vi "AeroQuadConfigurator.vi"() -> ()   [LabVIEW 2010] (continued)
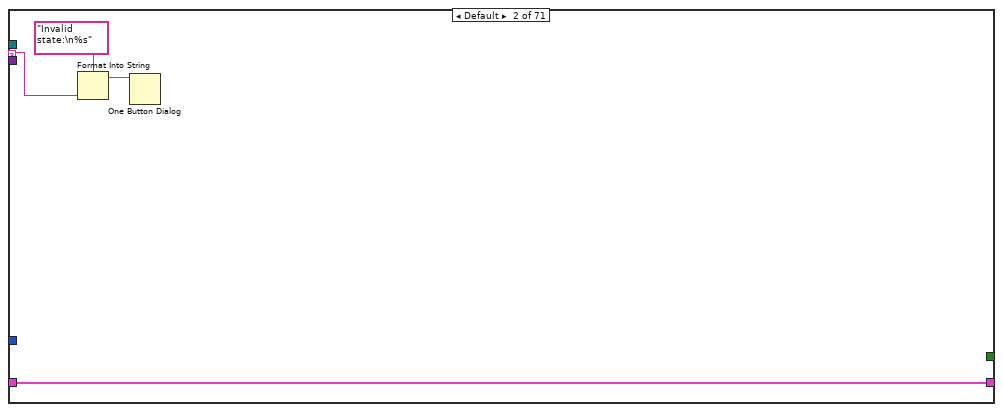
[diagram p3: hidden frame]
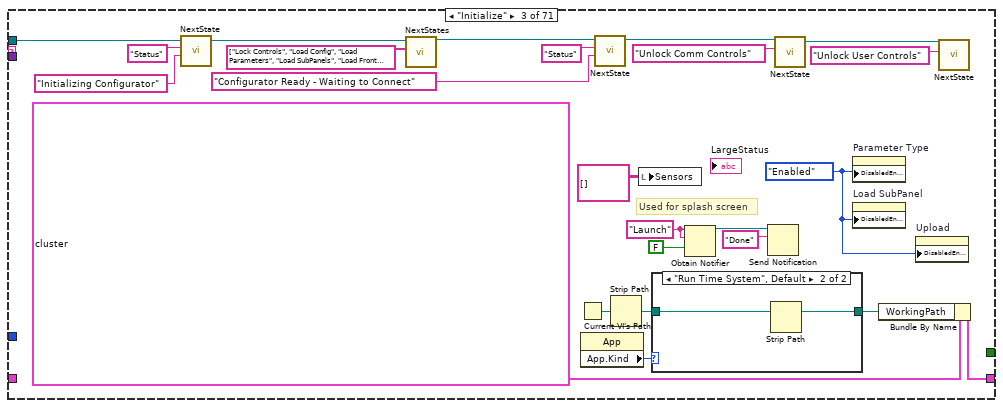
[diagram p4: hidden frame]
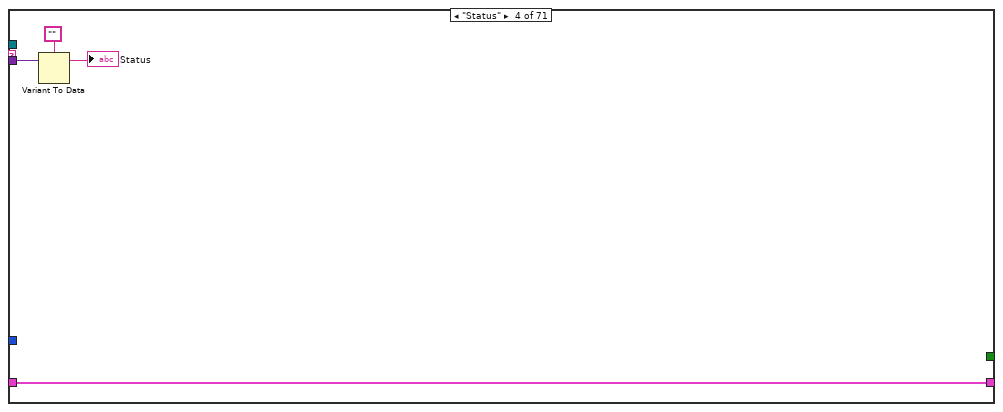
[diagram p6: hidden frame]
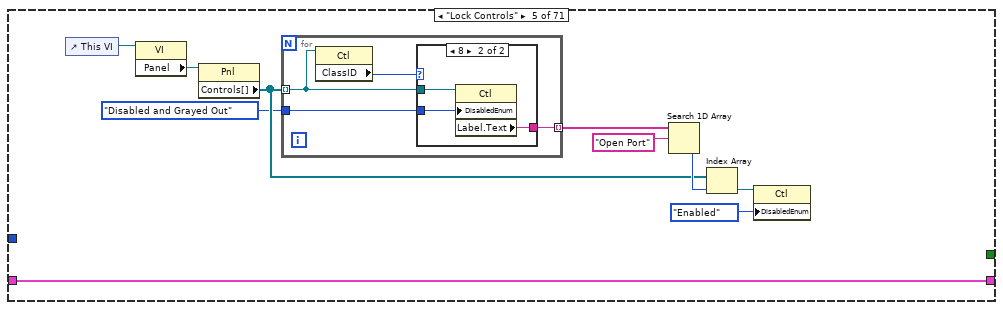
[diagram p7: hidden frame]
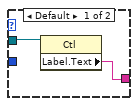
[diagram p8: hidden frame]
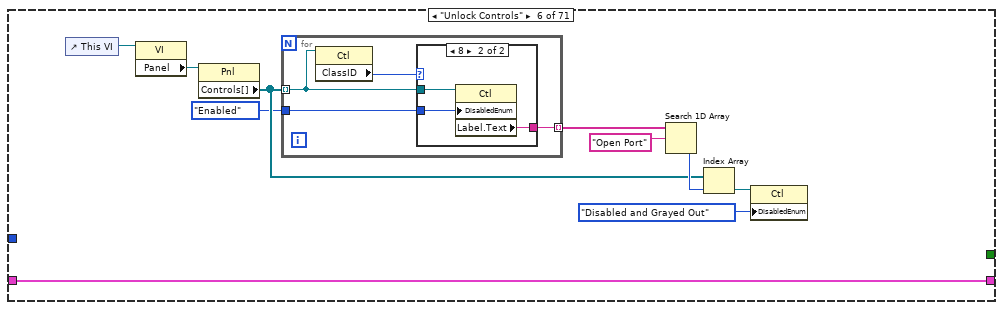
[diagram p9: hidden frame]
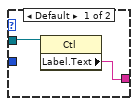
[diagram p10: hidden frame]
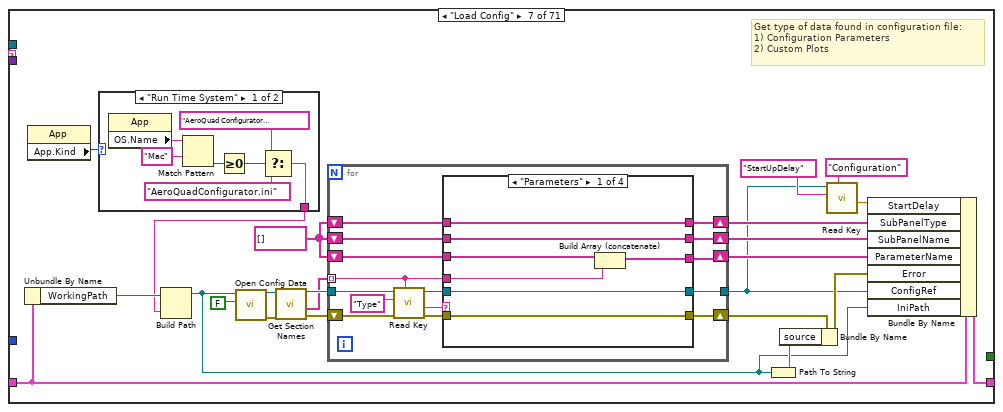
[diagram p11: hidden frame]
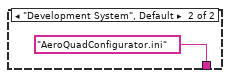
[diagram p12: hidden frame]
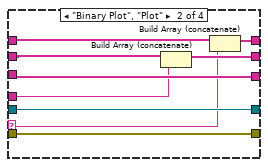
[diagram p13: hidden frame]
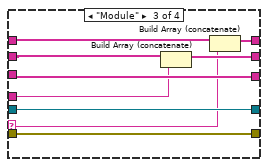
[diagram p14: hidden frame]
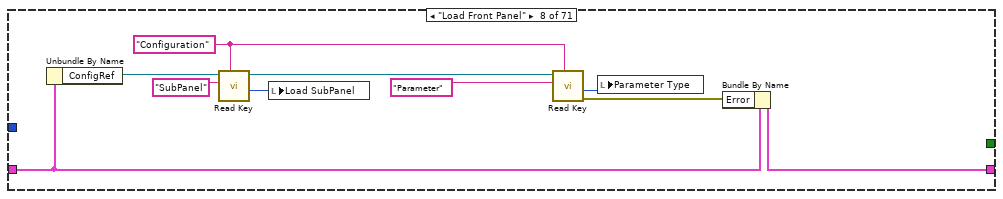
[diagram p16: hidden frame]
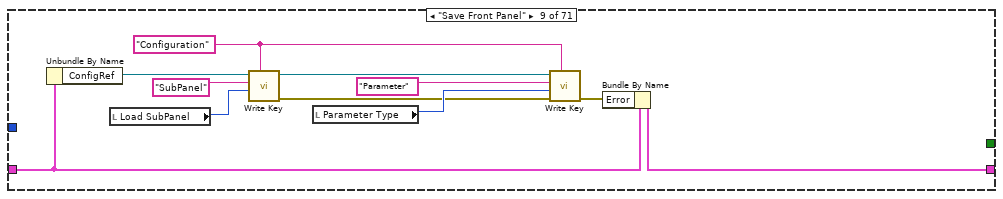
[diagram p17: hidden frame]
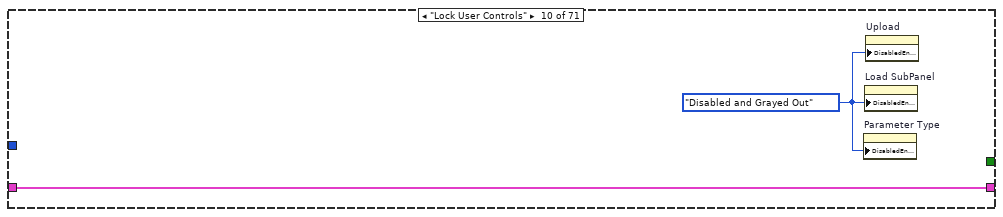
[diagram p18: hidden frame]
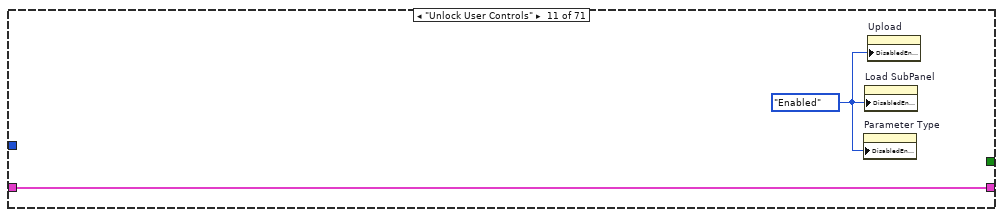
[diagram p19: hidden frame]
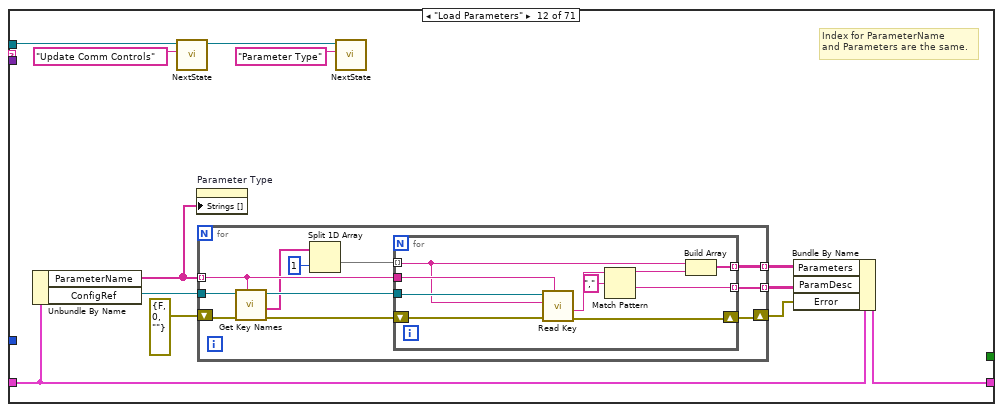
[diagram p20: hidden frame]
            n620 = call "RemoveTrailingComma.vi"("Input String"=w1295) -> ("Output String"=w1296:string)  [unwired: 8 in]
            n621 = Spreadsheet String To Array(delimiter (Tab)=",", format string="%s", spreadsheet string=w1296, array type (2D Dbl)=0) -> (array=w1301:i32[][])
            n622 = call "NextState.vi"("Data"=w1301, "State"="Update", "Queue In"=w1300) -> ()  [unwired: 7 in, 2 out]
            n623 = case shown="True" w1297 {
              tunnel: w1298 -> [_ w1312]
              tunnel: w1295 -> [_ w1311]
              frame False {
              }
              frame True {
                n624 = call "NextState.vi"("Data"=w1311, "State"="Read", "Queue In"=w1312) -> ()  [unwired: 7 in, 2 out]
              }
            }
          }
        }
      }
      frame "Read Serial Monitor Data" {
        n625 = Unbundle By Name(w1319) -> ("Logger"=w1314:bool, "DebugLogger"=w1313:refnum<queue>, "SubPanelQueue"=w1317:refnum<queue>, "COM Port"=w1320:refnum<visa-resource-name>, "Connected"=w1316:bool)
        n626 = case shown="True" w1316 {
          tunnel: w1320 -> [_ w1332]
          tunnel: w1319 -> [w1321 w1328]
          tunnel: [w1321 w1327] -> w1318
          tunnel: w1317 -> [_ w1331]
          tunnel: w1315 -> [_ w1325]
          tunnel: w1314 -> [_ w1324]
          tunnel: w1313 -> [_ w1323]
          frame False {
          }
          frame True {
            n627 = VISA Read(VISA resource name=w1332, byte count=u32 1024) -> (read buffer=w1322:string, error out=w1329:errorcluster)  [unwired: 1 in, 2 out]
            n628 = case shown="True" w1324 {
              tunnel: w1323 -> [_ w1336]
              tunnel: w1322 -> [_ w1335]
              frame False {
              }
              frame True {
                n629 = call "NextState.vi"("Data"=w1335, "State"="Read", "Queue In"=w1336) -> ()  [unwired: 7 in, 2 out]
              }
            }
            n630 = Unbundle By Name(w1329) -> ("code"=w1330:i32)
            n631 = case shown="0" w1330 {
              tunnel: w1322 -> [_ _ w1342]
              tunnel: w1331 -> [_ _ w1344]
              tunnel: [w1337 w1338 w1343] -> w1326
              tunnel: w1329 -> [w1337 w1339 _]
              tunnel: w1325 -> [_ _ w1341]
              frame Default {
              }
              frame -1073807339, -1073807252, 56 {
                n632 = call <vilib>:"Clear Errors.vi"("error in (no error)"=w1339) -> ("error out"=w1338:errorcluster)  [unwired: 6 out]
              }
              frame 0 {
                n633 = call "NextState.vi"("Data"=w1342, "State"="Update", "Queue In"=w1344) -> ("Error Out"=w1343:errorcluster)  [unwired: 7 in, 1 out]
                n634 = call "NextState.vi"("State"="Read Serial Monitor Data", "Queue In"=w1341) -> ()  [unwired: 8 in, 2 out]
              }
            }
            n635 = Bundle By Name(cluster=w1328, "Error"=w1326) -> (w1327:T2)
          }
        }
      }
      frame "Verify Upload" {
        n636 = Variant To Data(Variant=w1351, type="") -> (data=w1349:string)  [unwired: 1 in, 1 out]
        n637 = Unbundle By Name(w1354) -> ("Logger"=w1347:bool, "DebugLogger"=w1346:refnum<queue>, "COM Port"=w1355:refnum<visa-resource-name>, "Connected"=w1352:bool)
        n638 = case shown="True" w1352 {
          tunnel: w1355 -> [_ w1374]
          tunnel: w1354 -> [w1356 w1373]
          tunnel: [w1356 w1372] -> w1353
          tunnel: w1349 -> [_ w1366]
          tunnel: w1348 -> [_ w1370]
          tunnel: w1347 -> [_ w1362]
          tunnel: w1346 -> [_ w1361]
          frame False {
          }
          frame True {
            n639 = call "RemoveTrailingComma.vi"("Input String"=w1366) -> ("Output String"=w1363:string)  [unwired: 8 in]
            n640 = VISA Read(VISA resource name=w1374, byte count=u32 1024) -> (VISA resource name out=w1369:refnum<visa-resource-name>, read buffer=w1359:string, error out=w1367:errorcluster)  [unwired: 1 in, 1 out]
            n641 = case shown="True" w1362 {
              selector: w1362 -> [_ w1378]
              tunnel: w1361 -> [w1376 w1381]
              tunnel: w1359 -> [_ w1380]
              tunnel: [_ w1378] -> w1358
              tunnel: [w1376 w1377] -> w1357
              frame False {
              }
              frame True {
                n642 = call "NextState.vi"("Data"=w1380, "State"="Read", "Queue In"=w1381) -> ("Queue Out"=w1377:refnum<queue>)  [unwired: 7 in, 1 out]
              }
            }
            n643 = call "RemoveTrailingComma.vi"("Input String"=w1359) -> ("Output String"=w1360:string)  [unwired: 8 in]
            n644 = call "ConvertNumericString.vi"("Input"=w1363) -> ("Output"=w1365:string)  [unwired: 8 in]
            n645 = call "ConvertNumericString.vi"("Input"=w1360) -> ("Output"=w1364:string)  [unwired: 8 in]
            n646 = Equal?(x=w1365, y=w1364) -> (x = y?=w1371:bool)
            n647 = case shown="False" w1371 {
              tunnel: w1360 -> [w1387 w1393]
              tunnel: w1363 -> [w1388 _]
              tunnel: w1370 -> [w1382 w1401]
              tunnel: w1369 -> [_ w1404]
              tunnel: [w1385 w1403] -> w1368
              tunnel: w1367 -> [w1385 w1402]
              tunnel: w1358 -> [_ w1398]
              tunnel: w1357 -> [_ w1397]
              frame False {
                n648 = Format Into String(format string="Parameter update was not successful.\nExpected Response:\n%s\n\nTry Again?\nReceived Response:\n%s", w1388, w1387) -> (resulting string=w1386:string)  [unwired: 2 in, 1 out]
                n649 = Two Button Dialog(message=w1386, 2:"Retry" ("T button name (\"OK\")")) -> (T button?=w1383:bool)  [unwired: 1 in]
                n650 = case shown="False" w1383 {
                  tunnel: w1382 -> [_ w1392]
                  frame False {
                    w1390 = T3."Enabled" ("Disabled")
                    n651 = property on="Parameter Type" class="Ring (strict)"("DisabledEnum"=w1390) -> ()  [unwired: 2 in, 2 out]
                    n652 = property on="Upload" class="Bool"("DisabledEnum"=w1390) -> ()  [unwired: 2 in, 2 out]
                  }
                  frame True {
                    n653 = call "PriorityState.vi"("State"="Retry Upload", "Queue In"=w1392) -> ()  [unwired: 8 in, 2 out]
                  }
                }
              }
              frame True {
                w1396 = "W" ("write buffer")
                n654 = call "PriorityState.vi"("Data"="Upload successful!", "State"="Status", "Queue In"=w1401) -> ("Queue Out"=w1395:refnum<queue>)  [unwired: 7 in, 1 out]
                n655 = case shown="True" w1398 {
                  tunnel: w1397 -> [_ w1407]
                  tunnel: w1396 -> [_ w1405]
                  frame False {
                  }
                  frame True {
                    n656 = call "PriorityState.vi"("Data"=w1405, "State"="Write", "Queue In"=w1407) -> ()  [unwired: 7 in, 2 out]
                  }
                }
                n657 = call "NextState.vi"("Data"=w1393, "State"="Easy Update", "Queue In"=w1395) -> ()  [unwired: 7 in, 2 out]
                n658 = VISA Write(VISA resource name=w1404, write buffer=w1396, error in (no error)=w1402) -> (error out=w1403:errorcluster)  [unwired: 2 out]
              }
            }
            n659 = Bundle By Name(cluster=w1373, "Error"=w1368, "previousValid"=w1366) -> (w1372:T2)
          }
        }
      }
      frame "Retry Upload" {
        n660 = Unbundle By Name(w1421) -> ("oldCmd"=w1419:string, "oldTelem"=w1408:string, "previousValid"=w1409:string)
        n661 = disable-structure shown="Disabled" {
          disable-tunnel: w1415 -> [w1423 w1424]
          disable-tunnel: [w1422 w1424] -> w1414
          frame Disabled {
            n662 = Flush Queue(queue=w1423) -> (queue out=w1422:refnum<queue>)  [unwired: 1 in, 2 out]
          }
          frame Enabled {
          }
        }
        n663 = call "NextState.vi"("Data"=w1419, "State"="Send Command", "Queue In"=w1414) -> ("Queue Out"=w1417:refnum<queue>)  [unwired: 7 in, 1 out]
        n664 = call "NextState.vi"("State"="Delay SubPanel", "Queue In"=w1417) -> ("Queue Out"=w1412:refnum<queue>)  [unwired: 8 in, 1 out]
        n665 = call "NextState.vi"("Data"=w1408, "State"="Request Telemetry", "Queue In"=w1412) -> ("Queue Out"=w1411:refnum<queue>)  [unwired: 7 in, 1 out]
        n666 = call "NextState.vi"("Data"=w1409, "State"="Verify Upload", "Queue In"=w1411) -> ("Queue Out"=w1413:refnum<queue>)  [unwired: 7 in, 1 out]
        n667 = disable-structure shown="Disabled" {
          disable-tunnel: w1413 -> [w1426 _]
          frame Disabled {
            n668 = call "NextState.vi"("State"="Update Parameter", "Queue In"=w1426) -> ()  [unwired: 8 in, 2 out]
          }
          frame Enabled {
          }
        }
      }
      frame "--- File Operations ---" {
      }
      frame "File Open" {
        n669 = call "File Dialog"("prompt"="Select AeroQuad Config File", "pattern (all files)"="*.aq", "pattern label"="AeroQuad Config") -> ("selected path"=w1432:path, "cancelled"=w1428:bool)  [unwired: 9 in, 2 out]
        n670 = case shown="False" w1428 {
          tunnel: w1432 -> [w1460 _]
          tunnel: w1430 -> [w1459 _]
          tunnel: w1431 -> [w1442 _]
          tunnel: w1430 -> [w1446 w1489]
          tunnel: [w1445 w1489] -> w1429
          frame False {
            w1436 = 0
            n671 = Unbundle By Name(w1459) -> ("ParameterName"=w1453:string[], "Parameters"=w1452:string[][][])
            n672 = Flush Queue(queue=w1442) -> (queue out=w1438:refnum<queue>)  [unwired: 1 in, 2 out]
            n673 = call <vilib>:"Open Config Data.vi"("configuration file path"=w1460) -> ("error out"=w1457:errorcluster, "refnum"=w1458:T1)  [unwired: 8 in, 1 out]
            n674 = call <vilib>:"Get Section Names.vi"("error in (no error)"=w1457, "refnum"=w1458) -> ("error out"=w1455:errorcluster, "section names"=w1454:string[], "refnum out"=w1456:T1)  [unwired: 7 in]
            n675 = for {
              tunnel: w1456 -> [w1474]
              shift-right: [w1462] -> w1449
              shift-left: w1455 -> [w1473]
              tunnel: w1454 -> [w1468] mode=indexing
              tunnel: w1453 -> [w1475]
              shift-right: [w1464] -> w1451
              shift-left: w1452 -> [w1466]
              tunnel: [w1461] -> w1448
              n676 = call <vilib>:"Get Key Names.vi"("section"=w1468, "error in (no error)"=w1473, "refnum"=w1474) -> ("error out"=w1463:errorcluster, "key names"=w1469:string[], "refnum out"=w1470:T1)  [unwired: 5 in, 1 out]
              n677 = Search 1D Array(1D array=w1475, element=w1468) -> (index of element=w1465:i32)  [unwired: 1 in]
              n678 = Index Array(array=w1466, index (dim 0)=w1465) -> (element=w1471:string[][])  [unwired: 2 in]
              n679 = Index Array(array=w1471, index (col)=0 ("disabled index (col)")) -> (element=w1467:string[])  [unwired: 1 in]
              n680 = for {
                tunnel: w1470 -> [w1488]
                tunnel: w1469 -> [w1485] mode=indexing
                tunnel: w1468 -> [w1487]
                tunnel: w1467 -> [w1486]
                shift-right: [w1479] -> w1464
                shift-left: w1466 -> [w1484]
                tunnel: w1465 -> [w1483]
                shift-right: [w1477] -> w1462
                shift-left: w1463 -> [w1478]
                tunnel: [w1476] -> w1461
                n681 = call-poly <vilib>:"Read Key.vi"("section"=w1487, "error in (no error)"=w1478, "key"=w1485, "refnum"=w1488) -> ("error out"=w1477:errorcluster, "value"=w1480:string, "refnum out"=w1476:T1)  [unwired: 4 in, 1 out]
                n682 = Search 1D Array(1D array=w1486, element=w1485) -> (index of element=w1481:i32)  [unwired: 1 in]
                n683 = Replace Array Subset(array=w1484, new element=w1480, index (dim 0)=w1483, index (dim 1)=w1481, index (dim 2)=1 ("disabled index (col)")) -> (w1479:string[][][])
              }
            }
            n684 = call "NextState.vi"("State"="Clear Serial Comm", "Queue In"=w1438) -> ("Queue Out"=w1441:refnum<queue>)  [unwired: 8 in, 1 out]
            n685 = call "NextState.vi"("State"="Default Timeout", "Queue In"=w1441) -> ("Queue Out"=w1439:refnum<queue>)  [unwired: 8 in, 1 out]
            n686 = call "NextState.vi"("State"="Parameter Type", "Queue In"=w1439) -> ("Queue Out"=w1443:refnum<queue>)  [unwired: 8 in, 1 out]
            n687 = call <vilib>:"Close Config Data.vi"("error in (no error)"=w1449, "refnum"=w1448) -> ("error out"=w1447:errorcluster)  [unwired: 8 in, 1 out]
            n688 = Bundle By Name(cluster=w1446, "Error"=w1447, "Parameters"=w1451) -> (w1445:T2)
            n689 = property on="Parameter Type" class="Ring (strict)"("Value"=w1436) -> ()  [unwired: 2 in, 2 out]
            n690 = call "NextState.vi"("Data"=w1436, "State"="File Upload", "Queue In"=w1443) -> ()  [unwired: 7 in, 2 out]
          }
          frame True {
          }
        }
      }
      frame "File Next" {
        n691 = Variant To Data(Variant=w1494, type=0) -> (data=w1491:i32)  [unwired: 1 in, 1 out]
        n692 = property on="Parameter Type" class="Ring (strict)"() -> ("NumItems"=w1496:u32)  [unwired: 2 in, 2 out]
        n693 = Increment(x=w1491) -> (x+1=w1490:i32)
        n694 = Less?(x=w1490, y=w1496) -> (x < y?=w1495:bool)
        n695 = case shown="True" w1495 {
          tunnel: w1490 -> [_ w1503]
          tunnel: w1492 -> [w1502 w1506]
          frame False {
            n696 = call "NextState.vi"("Data"="Finished loading AeroQuad configuration file." ("State"), "State"="Status", "Queue In"=w1502) -> ("Queue Out"=w1498:refnum<queue>)  [unwired: 7 in, 1 out]
            n697 = call "NextState.vi"("State"="Load SubPanel", "Queue In"=w1498) -> ()  [unwired: 8 in, 2 out]
          }
          frame True {
            n698 = local write "Parameter Type"(w1503) -> ()
            n699 = call "NextState.vi"("State"="Parameter Type", "Queue In"=w1506) -> ("Queue Out"=w1504:refnum<queue>)  [unwired: 8 in, 1 out]
            n700 = call "NextState.vi"("Data"=w1503, "State"="File Upload", "Queue In"=w1504) -> ()  [unwired: 7 in, 2 out]
          }
        }
      }
      frame "File Upload" {
        n701 = Variant To Data(Variant=w1509, type=0) -> (data=w1508:i32)  [unwired: 1 in, 1 out]
        n702 = Unbundle By Name(w1557) -> ("Parameters"=w1532:string[][][])
        n703 = local read "Parameter Check"() -> (w1554:string[][])
        n704 = Index Array(array=w1554, index (col)=0 ("disabled index (col)")) -> (element=w1537:string[])  [unwired: 1 in]
        n705 = Index Array(array=w1532, index (dim 0)=w1508, index (dim 2)=0 ("disabled index (row)")) -> (element=w1545:string[])  [unwired: 1 in]
        n706 = Array To Spreadsheet String(delimiter (Tab)=";", array=w1537, 3:"%s" ("format string")) -> (spreadsheet string=w1527:string)
        n707 = Search 1D Array(1D array=w1545, element="Command") -> (index of element=w1534:i32)  [unwired: 1 in]
        n708 = Match Pattern(string=w1527, regular expression=";;") -> (before substring=w1529:string)  [unwired: 4 out]
        n709 = Index Array(array=w1532, index (dim 0)=w1508, index (dim 1)=w1534, index (dim 2)=1 ("disabled index (col)")) -> (element=w1548:string)
        n710 = Match Pattern(string=w1529, regular expression="\r\n") -> (before substring=w1538:string)  [unwired: 4 out]
        n711 = Format Into String(format string="%s%s;", w1548, w1538) -> (resulting string=w1547:string)  [unwired: 2 in, 1 out]
        n712 = Array To Spreadsheet String(delimiter (Tab)=",", array=w1537, 3:"%s" ("format string")) -> (spreadsheet string=w1525:string)
        n713 = call "NextState.vi"("Data"=w1547, "State"="Send Command", "Queue In"=w1522) -> ("Queue Out"=w1543:refnum<queue>)  [unwired: 7 in, 1 out]
        n714 = Search 1D Array(1D array=w1545, element="Telemetry") -> (index of element=w1531:i32)  [unwired: 1 in]
        n715 = Match Pattern(string=w1525, regular expression=",,") -> (before substring=w1526:string)  [unwired: 4 out]
        n716 = Index Array(array=w1532, index (dim 0)=w1508, index (dim 1)=w1531, index (dim 2)=1 ("disabled index (col)")) -> (element=w1513:string)
        n717 = call "NextState.vi"("Data"=w1513, "State"="Request Telemetry", "Queue In"=w1543) -> ("Queue Out"=w1542:refnum<queue>)  [unwired: 7 in, 1 out]
        n718 = Match Pattern(string=w1526, regular expression="\r\n") -> (before substring=w1521:string)  [unwired: 4 out]
        n719 = property on="Parameter Type" class="Ring (strict)"() -> ("Strings []"=w1515:string[])  [unwired: 2 in, 2 out]
        n720 = call "NextState.vi"("Data"=w1521, "State"="Verify Upload", "Queue In"=w1542) -> ("Queue Out"=w1520:refnum<queue>)  [unwired: 7 in, 1 out]
        n721 = call "NextState.vi"("State"="Update Parameter", "Queue In"=w1520) -> ("Queue Out"=w1519:refnum<queue>)  [unwired: 8 in, 1 out]
        n722 = Index Array(array=w1515, index=w1508) -> (element=w1514:string)
        n723 = Format Into String(format string="Uploaded %s parameters.", w1514) -> (resulting string=w1516:string)  [unwired: 2 in, 1 out]
        n724 = call "NextState.vi"("Data"=w1516, "State"="Status", "Queue In"=w1519) -> ("Queue Out"=w1512:refnum<queue>)  [unwired: 7 in, 1 out]
        n725 = call "NextState.vi"("Data"=w1508, "State"="File Next", "Queue In"=w1512) -> ()  [unwired: 7 in, 2 out]
      }
      frame "File Save" {
        n726 = call "File Dialog2"("prompt"="Save AeroQuad Config File", "pattern (all files)"="*.aq", "pattern label"="AeroQuad Config") -> ("selected path"=w1558:path, "cancelled"=w1559:bool)  [unwired: 9 in, 2 out]
        n727 = case shown="False" w1559 {
          tunnel: w1563 -> [w1569 _]
          tunnel: w1558 -> [w1564 _]
          frame False {
            n728 = Unbundle By Name(w1569) -> ("ParameterName"=w1570:string[], "Parameters"=w1571:string[][][])
            n729 = property on="Parameter Type" class="Ring (strict)"() -> ("NumItems"=w1572:u32)  [unwired: 2 in, 2 out]
            n730 = call <vilib>:"Open Config Data.vi"("configuration file path"=w1564) -> ("error out"=w1568:errorcluster, "refnum"=w1565:T1)  [unwired: 8 in, 1 out]
            n731 = for {
              N: w1572 -> [_]
              tunnel: w1571 -> [w1582]
              tunnel: w1570 -> [w1577] mode=indexing
              shift-right: [w1575] -> w1567
              shift-left: w1568 -> [w1576]
              tunnel: [w1574] -> w1566
              tunnel: w1565 -> [w1573]
              i -> [w1581]
              n732 = Index Array(array=w1582, index (dim 0) #1=w1581, index (dim 0) #2=w1581, index (dim 2) #2=0 ("disabled index (col)")) -> (element #1=w1578:string[][], element #2=w1579:string[])  [unwired: 3 in]
              n733 = for {
                tunnel: w1579 -> [w1589] mode=indexing
                tunnel: w1578 -> [w1588] mode=indexing
                tunnel: w1577 -> [w1587]
                shift-right: [w1585] -> w1575
                shift-left: w1576 -> [w1586]
                tunnel: [w1584] -> w1574
                tunnel: w1573 -> [w1583]
                n734 = case shown="Default" w1589 {
                  tunnel: w1588 -> [w1596 _]
                  tunnel: w1587 -> [w1597 _]
                  tunnel: w1586 -> [w1593 w1599]
                  tunnel: [w1592 w1599] -> w1585
                  tunnel: [w1591 w1598] -> w1584
                  tunnel: w1583 -> [w1590 w1598]
                  frame Default {
                    n735 = Index Array(array=w1596) -> (element #1=w1595:string, element #2=w1594:string)  [unwired: 2 in]
                    n736 = call-poly <vilib>:"Write Key.vi"("section"=w1597, "error in (no error)"=w1593, "value"=w1594, "key"=w1595, "refnum"=w1590) -> ("error out"=w1592:errorcluster, "refnum out"=w1591:T1)  [unwired: 4 in, 1 out]
                  }
                  frame "Command", "Telemetry" {
                  }
                }
              }
            }
            n737 = call <vilib>:"Close Config Data.vi"("error in (no error)"=w1567, "refnum"=w1566) -> ()  [unwired: 8 in, 2 out]
          }
          frame True {
          }
        }
      }
      frame "--- Calibrations ---" {
      }
      frame "Store Calibration" {
        w1602 = "Calibrations" ("section")
        n738 = Unbundle By Name(w1624) -> ("IniPath"=w1614:path, "ConfigRef"=w1611:T1)
        n739 = Variant To Data(Variant=w1626, type=w1625) -> (data=w1610:string)  [unwired: 1 in, 1 out]
        n740 = String Subset(string=w1610, length (rest)=1 ("length (rest)")) -> (substring=w1607:string)  [unwired: 1 in]
        n741 = call <vilib>:"Get Key Names.vi"("section"=w1602, "refnum"=w1611) -> ("key names"=w1608:string[], "refnum out"=w1604:T1)  [unwired: 6 in, 2 out]
        n742 = for {
          tunnel: w1608 -> [w1639] mode=indexing
          tunnel: w1607 -> [w1641]
          tunnel: [w1640] -> w1606
          tunnel: [w1639] -> w1605
          tunnel: [w1638] -> w1601
          stop <- w1640 stop-if-true
          n743 = String Subset(string=w1639, length (rest)=1 ("length (rest)")) -> (substring=w1638:string)  [unwired: 1 in]
          n744 = Equal?(x=w1641, y=w1638) -> (x = y?=w1640:bool)
        }
        n745 = case shown="True" w1606 {
          tunnel: w1605 -> [_ w1632]
          tunnel: w1604 -> [w1627 w1631]
          tunnel: [w1627 w1630] -> w1603
          tunnel: w1602 -> [_ w1629]
          tunnel: w1601 -> [_ w1628]
          frame False {
          }
          frame True {
            n746 = case shown="\"K\", \"M\"" w1628 {
              tunnel: w1632 -> [_ w1637]
              tunnel: w1631 -> [w1633 w1636]
              tunnel: [w1633 w1635] -> w1630
              tunnel: w1629 -> [_ w1634]
              frame Default {
              }
              frame "K", "M" {
                n747 = call <vilib>:"Remove Key.vi"("section"=w1634, "key"=w1637, "refnum"=w1636) -> ("refnum out"=w1635:T1)  [unwired: 6 in, 2 out]
              }
            }
          }
        }
        n748 = Match Pattern(string=w1610, regular expression=";") -> (before substring=w1621:string, match substring=w1620:string, after substring=w1618:string)  [unwired: 1 in, 1 out]
        n749 = Concatenate Strings(w1621, w1620) -> (w1619:string)
        n750 = call-poly <vilib>:"Write Key.vi"("section"=w1602, "value"=w1618, "key"=w1619, "refnum"=w1603) -> ("error out"=w1616:errorcluster, "refnum out"=w1617:T1)  [unwired: 5 in, 1 out]
        n751 = call <vilib>:"Close Config Data.vi"("error in (no error)"=w1616, "refnum"=w1617) -> ("error out"=w1615:errorcluster)  [unwired: 8 in, 1 out]
        n752 = call <vilib>:"Open Config Data.vi"("error in (no error)"=w1615, "configuration file path"=w1614) -> ("error out"=w1613:errorcluster, "refnum"=w1612:T1)  [unwired: 7 in, 1 out]
        n753 = Bundle By Name(cluster=w1624, "ConfigRef"=w1612, "Error"=w1613) -> (w1623:T2)
      }
      frame "Recall Calibrations" {
        n754 = Variant To Data(Variant=w1654, type=w1653) -> (data=w1652:string)  [unwired: 1 in, 1 out]
        n755 = Unbundle By Name(w1651) -> ("ConfigRef"=w1650:T1)
        n756 = call "NextState.vi"("Data"="Recalling calibrations..." ("State"), "State"="Status", "Queue In"=w1648) -> ("Queue Out"=w1647:refnum<queue>)  [unwired: 7 in, 1 out]
        n757 = case shown="Default" w1652 {
          selector: w1652 -> [w1656 _]
          tunnel: w1650 -> [w1667 w1701]
          tunnel: w1647 -> [w1657 w1695]
          tunnel: [w1658 w1698] -> w1643
          tunnel: [w1655 w1693] -> w1644
          frame Default {
            w1661 = "Calibrations" ("section")
            n758 = call-poly <vilib>:"Read Key.vi"("section"="Initial Setup", "key"=w1656, "refnum"=w1667) -> ("value"=w1664:string, "refnum out"=w1665:T1)  [unwired: 5 in, 2 out]
            n759 = call <vilib>:"Get Key Names.vi"("section"=w1661, "refnum"=w1665) -> ("key names"=w1663:string[], "refnum out"=w1662:T1)  [unwired: 6 in, 2 out]
            n760 = for {
              tunnel: w1664 -> [w1678]
              tunnel: w1663 -> [w1676] mode=indexing
              tunnel: w1662 -> [w1675]
              tunnel: [w1674] -> w1660 mode=indexing
              tunnel: w1661 -> [w1673]
              tunnel: w1657 -> [w1672]
              n761 = String Subset(string=w1676, length (rest)=1 ("length (rest)")) -> (substring=w1679:string)  [unwired: 1 in]
              n762 = Equal?(x=w1679, y=w1678) -> (x = y?=w1677:bool)
              n763 = case shown="True" w1677 {
                selector: w1677 -> [w1681 w1692]
                tunnel: w1676 -> [_ w1689]
                tunnel: w1675 -> [_ w1691]
                tunnel: [w1681 w1692] -> w1674
                tunnel: w1673 -> [_ w1690]
                tunnel: w1672 -> [_ w1687]
                frame False {
                }
                frame True {
                  n764 = call-poly <vilib>:"Read Key.vi"("section"=w1690, "key"=w1689, "refnum"=w1691) -> ("value"=w1688:string)  [unwired: 5 in, 3 out]
                  n765 = Concatenate Strings(w1689, w1688) -> (w1685:string)
                  n766 = call "NextState.vi"("Data"=w1685, "State"="Send Command", "Queue In"=w1687) -> ("Queue Out"=w1683:refnum<queue>)  [unwired: 7 in, 1 out]
                  n767 = call "NextState.vi"("Data"=100, "State"="Delay", "Queue In"=w1683) -> ()  [unwired: 7 in, 2 out]
                }
              }
            }
            n768 = Or Array Elements(Boolean array=w1660) -> (logical OR=w1659:bool)
            n769 = case shown="True" w1659 {
              tunnel: w1657 -> [w1668 w1671]
              tunnel: [w1668 w1671] -> w1658
              tunnel: w1656 -> [_ _]
              tunnel: ["No calibrations found." ("State") " Calibration Recalled" ("State")] -> w1655
              frame False {
              }
              frame True {
              }
            }
          }
          frame "All" {
            w1699 = "Calibrations" ("section")
            n770 = call <vilib>:"Get Key Names.vi"("section"=w1699, "refnum"=w1701) -> ("key names"=w1697:string[], "refnum out"=w1700:T1)  [unwired: 6 in, 2 out]
            n771 = for {
              tunnel: w1700 -> [w1721]
              tunnel: w1699 -> [w1720]
              tunnel: w1697 -> [w1712] mode=indexing
              tunnel: w1695 -> [w1719]
              tunnel: [w1713] -> w1694
              n772 = call-poly <vilib>:"Read Key.vi"("section"=w1720, "key"=w1712, "refnum"=w1721) -> ("value"=w1717:string)  [unwired: 5 in, 3 out]
              n773 = Match Pattern(string=w1712, regular expression="K") -> (offset past match=w1710:i32)  [unwired: 1 in, 3 out]
              n774 = Greater Or Equal To 0?(x=w1710) -> (x >= 0?=w1708:bool)
              n775 = Concatenate Strings(w1712, w1717) -> (w1716:string)
              n776 = call "NextState.vi"("Data"=w1716, "State"="Send Command", "Queue In"=w1719) -> ("Queue Out"=w1715:refnum<queue>)  [unwired: 7 in, 1 out]
              n777 = Select(t=1500, s=w1708, f=300) -> (s? t:f=w1706:i32)
              n778 = call "NextState.vi"("Data"=w1706, "State"="Delay", "Queue In"=w1715) -> ("Error Out"=w1713:errorcluster)  [unwired: 7 in, 1 out]
            }
            n779 = Array Size(array=w1697) -> (size(s)=w1696:i32)
            n780 = case shown="Default" w1696 {
              tunnel: w1695 -> [w1703 w1705]
              tunnel: [w1703 w1705] -> w1698
              tunnel: w1694 -> [_ _]
              tunnel: ["No calibrations found." ("State") "Calibrations Recalled" ("State")] -> w1693
              frame 0 {
              }
              frame Default {
              }
            }
          }
        }
        n781 = call "NextState.vi"("Data"=w1644, "State"="Cleanup Recall", "Queue In"=w1643) -> ()  [unwired: 7 in, 2 out]
      }
      frame "Cleanup Recall" {
        n782 = Get Queue Status(queue=w1727) -> (queue out=w1723:refnum<queue>, elements=w1726:cluster{"State":string, "Data":variant}[])  [unwired: 2 in, 6 out]
        n783 = for "Fix later - currently nothing happens" {
          tunnel: w1726 -> [w1752] mode=indexing
          tunnel: [w1748] -> w1725 mode=indexing
          n784 = Unbundle By Name(w1752) -> ("State"=w1750:string)
          n785 = Match Pattern(string=w1750, regular expression="Recall Calibrations") -> (offset past match=w1749:i32)  [unwired: 1 in, 3 out]
          n786 = Greater Or Equal To 0?(x=w1749) -> (x >= 0?=w1748:bool)
        }
        n787 = Or Array Elements(Boolean array=w1725) -> (logical OR=w1724:bool)
        n788 = case shown="False" w1724 {
          tunnel: w1723 -> [w1738 w1747]
          tunnel: w1722 -> [w1730 w1745]
          frame False {
            n789 = call "NextState.vi"("Data"="W", "State"="Send Command", "Queue In"=w1738) -> ("Queue Out"=w1737:refnum<queue>)  [unwired: 7 in, 1 out]
            n790 = call "NextState.vi"("Data"=6000, "State"="Delay", "Queue In"=w1737) -> ("Queue Out"=w1736:refnum<queue>)  [unwired: 7 in, 1 out]
            n791 = call "NextState.vi"("Data"=w1730, "State"="Status", "Queue In"=w1736) -> ("Queue Out"=w1735:refnum<queue>)  [unwired: 7 in, 1 out]
            n792 = call "NextState.vi"("State"="Unlock User Controls", "Queue In"=w1735) -> ("Queue Out"=w1733:refnum<queue>)  [unwired: 8 in, 1 out]
            n793 = call "NextState.vi"("State"="Load SubPanel", "Queue In"=w1733) -> ()  [unwired: 8 in, 2 out]
          }
          frame True {
            n794 = call "NextState.vi"("Data"=w1745, "State"="Status", "Queue In"=w1747) -> ("Queue Out"=w1743:refnum<queue>)  [unwired: 7 in, 1 out]
            n795 = call "NextState.vi"("Data"=6000, "State"="Delay", "Queue In"=w1743) -> ()  [unwired: 7 in, 2 out]
          }
        }
      }
    }
  }
  n796 = while {
    tunnel: w6 -> [w1756]
    tunnel: w3 -> [w1755]
    tunnel: [w1753] -> w5
    stop <- w1754 stop-if-true
    n797 = event shown="[1] Menu Selection (User)" {
      selector: w1756 -> [_ _ _ _ _]
      dyn-events: [_ _ _ _ _] -> w1753
      timeout: _ -> [_ _ _ _ _]
      tunnel: w1755 -> [w1758 w1766 w1838 w1846 w1848]
      tunnel: [_ w1764 TRUE _ _] -> w1754
      event Value Change {
        # "If a control 's value has changed,\nit's name will be called as a state.\nIt will not go to a state if it has a * in it's name."
        n798 = event-data() -> ("CtlRef"=w1761:refnum<vi>)  [unwired: 1 in]
        n799 = property class="Ctl"(reference=w1761) -> ("Label.Text"=w1757:string)  [unwired: 1 in, 2 out]
        n800 = Match Pattern(string=w1757, regular expression="*") -> (offset past match=w1759:i32)  [unwired: 1 in, 3 out]
        n801 = case shown="..0" w1759 {
          tunnel: w1758 -> [_ w1763]
          tunnel: w1757 -> [_ w1762]
          frame Default {
          }
          frame ..0 {
            n802 = call "NextState.vi"("State"=w1762, "Queue In"=w1763) -> ()  [unwired: 8 in, 2 out]
          }
        }
      }
      event Menu Selection (User) {
        n803 = event-data() -> ("ItemTag"=w1765:string)  [unwired: 1 in]
        n804 = case shown="\"Connection Type:\"..\"Connection Type:z\"" w1765 {
          selector: w1765 -> [w1771 w1775 w1790 w1798 w1817 w1820]
          tunnel: w1766 -> [w1768 w1776 w1781 w1796 w1816 _]
          tunnel: [TRUE _ _ _ _ _] -> w1764
          frame "Exit" {
            n805 = call "NextState.vi"("State"="Save Front Panel", "Queue In"=w1768) -> ("Queue Out"=w1769:refnum<queue>)  [unwired: 8 in, 1 out]
            n806 = call "NextState.vi"("State"=w1771, "Queue In"=w1769) -> ()  [unwired: 8 in, 2 out]
          }
          frame Default {
            n807 = Match Pattern(string=w1775, regular expression=":") -> (before substring=w1773:string, after substring=w1772:string)  [unwired: 1 in, 2 out]
            n808 = call "NextState.vi"("Data"=w1772, "State"=w1773, "Queue In"=w1776) -> ()  [unwired: 7 in, 2 out]
          }
          frame "Recall Calibrations:".."Recall Calibrations:z" {
            n809 = Flush Queue(queue=w1781) -> (queue out=w1780:refnum<queue>)  [unwired: 1 in, 2 out]
            n810 = call "NextState.vi"("State"="Clear Serial Comm" ("GUI State"), "Queue In"=w1780) -> ("Queue Out"=w1779:refnum<queue>)  [unwired: 8 in, 1 out]
            n811 = call "NextState.vi"("State"="Lock User Controls" ("GUI State"), "Queue In"=w1779) -> ("Queue Out"=w1777:refnum<queue>)  [unwired: 8 in, 1 out]
            n812 = Match Pattern(string=w1790, regular expression=":") -> (before substring=w1788:string, after substring=w1786:string)  [unwired: 1 in, 2 out]
            n813 = Spreadsheet String To Array(delimiter (Tab)=",", format string="%s", spreadsheet string=w1786, array type (2D Dbl)=string[] []) -> (array=w1783:string[])
            n814 = for {
              tunnel: w1788 -> [w1794]
              tunnel: w1783 -> [w1793] mode=indexing
              tunnel: [w1792] -> _
              tunnel: w1777 -> [w1791]
              n815 = call "NextState.vi"("Data"=w1793, "State"=w1794, "Queue In"=w1791) -> ("Queue Out"=w1792:refnum<queue>)  [unwired: 7 in, 1 out]
            }
          }
          frame "Connection Type:".."Connection Type:z" {
            n816 = Current VI's Menubar() -> (w1800:refnum<k9>)
            n817 = Get Menu Item Info(7:"Connect" ("item tag"), 11:w1800) -> (3:w1803:refnum<k9>, 5:w1802:string[])  [unwired: 1 in, 5 out]
            n818 = for {
              tunnel: w1802 -> [w1807] mode=indexing
              tunnel: w1803 -> [w1810]
              tunnel: [w1808] -> w1804
              n819 = Set Menu Item Info(6:FALSE ("checked"), 7:w1807, 11:w1810) -> (3:w1808:refnum<k9>)  [unwired: 4 in, 1 out]
            }
            n820 = Set Menu Item Info(6:TRUE ("checked"), 7:w1798, 11:w1804) -> ()  [unwired: 4 in, 2 out]
            n821 = Match Pattern(string=w1798, regular expression=":") -> (before substring=w1797:string, after substring=w1795:string)  [unwired: 1 in, 2 out]
            n822 = call "NextState.vi"("Data"=w1795, "State"=w1797, "Queue In"=w1796) -> ()  [unwired: 7 in, 2 out]
            n823 = case shown="\"Modem\"" w1795 {
              frame Default {
              }
              frame "Modem" {
                n824 = One Button Dialog(message="Connection with the audio telemetry modem has been enabled.  In this mode, only Mission Planning features are enabled.") -> ()  [unwired: 1 in, 1 out]
              }
            }
          }
          frame "Communication Log" {
            n825 = Current VI's Menubar() -> (w1819:refnum<k9>)
            n826 = Get Menu Item Info(7:w1817, 11:w1819) -> (3:w1818:refnum<k9>, 4:w1815:bool)  [unwired: 1 in, 5 out]
            n827 = Not(x=w1815) -> (.not. x?=w1814:bool)
            n828 = Set Menu Item Info(6:w1814, 7:w1817, 11:w1818) -> ()  [unwired: 4 in, 2 out]
            n829 = Select(t="Open", s=w1814, f="Close") -> (s? t:f=w1811:string)
            n830 = call "NextState.vi"("Data"=w1811, "State"=w1817, "Queue In"=w1816) -> ()  [unwired: 7 in, 2 out]
          }
          frame "View:".."View:z" {
            n831 = Match Pattern(string=w1820, regular expression=":") -> (after substring=w1828:string)  [unwired: 1 in, 3 out]
            n832 = case shown="\"Basic\"" w1828 {
              tunnel: [809 ("Splitter Position") 1050 ("Splitter Position")] -> w1827
              frame "Advanced", Default {
              }
              frame "Basic" {
                (unwired) 1074 ("Splitter Position")
              }
            }
            n833 = disable-structure shown="Enabled" {
              disable-tunnel: w1827 -> [w1830 _]
              frame Disabled {
                n834 = property on="Splitter 3" class="Splitter"("Position"=w1830) -> ()  [unwired: 2 in, 2 out]
              }
              frame Enabled {
                n835 = One Button Dialog(message="Under Construction") -> ()  [unwired: 1 in, 1 out]
              }
            }
            n836 = Current VI's Menubar() -> (w1821:refnum<k9>)
            n837 = Get Menu Item Info(7:"View" ("item tag"), 11:w1821) -> (3:w1824:refnum<k9>, 5:w1823:string[])  [unwired: 1 in, 5 out]
            n838 = for {
              tunnel: w1823 -> [w1832] mode=indexing
              tunnel: w1824 -> [w1835]
              tunnel: [w1833] -> w1825
              n839 = Set Menu Item Info(6:FALSE ("checked"), 7:w1832, 11:w1835) -> (3:w1833:refnum<k9>)  [unwired: 4 in, 1 out]
            }
            n840 = Set Menu Item Info(6:TRUE ("checked"), 7:w1820, 11:w1825) -> ()  [unwired: 4 in, 2 out]
          }
        }
      }
      event Panel Close? {
        n841 = event-data() -> ()  [unwired: 1 in, 1 out]
        n842 = call "NextState.vi"("State"="Save Front Panel", "Queue In"=w1838) -> ("Queue Out"=w1839:refnum<queue>)  [unwired: 8 in, 1 out]
        n843 = call "NextState.vi"("State"="Exit", "Queue In"=w1839) -> ()  [unwired: 8 in, 2 out]
        n844 = event-data("Discard?"=TRUE) -> ()  [unwired: 1 in, 1 out]
      }
      event "Parameter Check": Mouse Down {
        n845 = event-data() -> ()  [unwired: 1 in, 1 out]
        n846 = property on="Parameter Check" class="Tbl (strict)"() -> ("EditPos"=w1847:T6)  [unwired: 2 in, 2 out]
        n847 = Unbundle By Name(w1847) -> ("Row"=w1844:i32)
        n848 = call "NextState.vi"("Data"=w1844, "State"="Update Tool Tip", "Queue In"=w1846) -> ()  [unwired: 7 in, 2 out]
      }
      event Key Down {
        n849 = event-data() -> ("Char"=w1849:i16)  [unwired: 1 in]
        n850 = case shown="9" w1849 {
          tunnel: w1848 -> [w1851 _]
          frame 9 {
            n851 = call "NextState.vi"("State"="Next Parameter", "Queue In"=w1851) -> ()  [unwired: 8 in, 2 out]
          }
          frame Default {
          }
        }
      }
    }
  }
  n852 = Unregister For Events(event registration refnum=w5) -> ()  [unwired: 1 in, 1 out]
